vi "UHR-Fleezers Control (host) - 10.7.vi"() -> ()   [LabVIEW 2010] (continued)
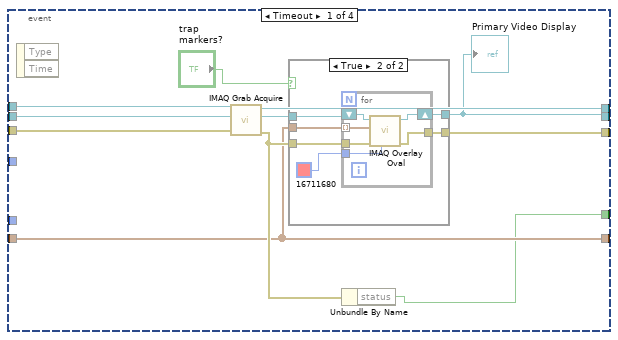
[diagram p2: hidden frame]
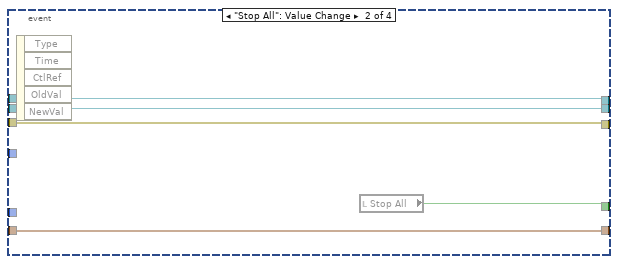
[diagram p4: hidden frame]
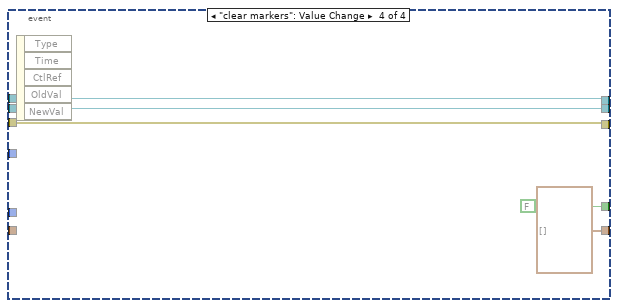
[diagram p6: hidden frame]
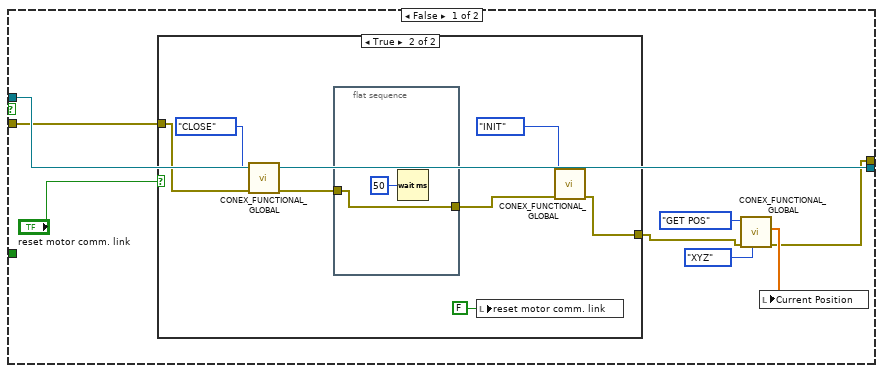
[diagram p8: hidden frame]
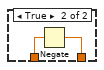
[diagram p12: hidden frame]
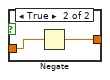
[diagram p13: hidden frame]
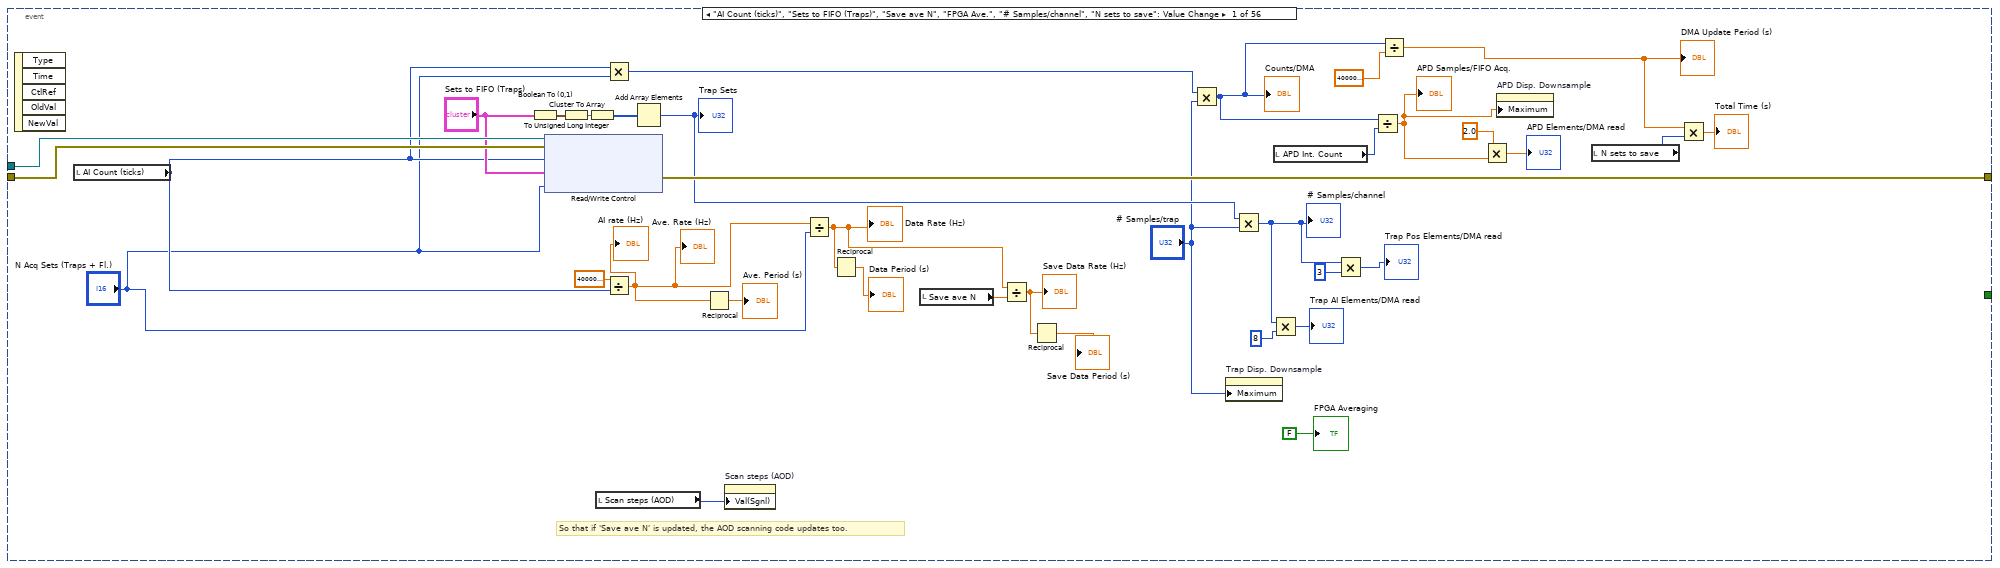
[diagram p14: hidden frame]
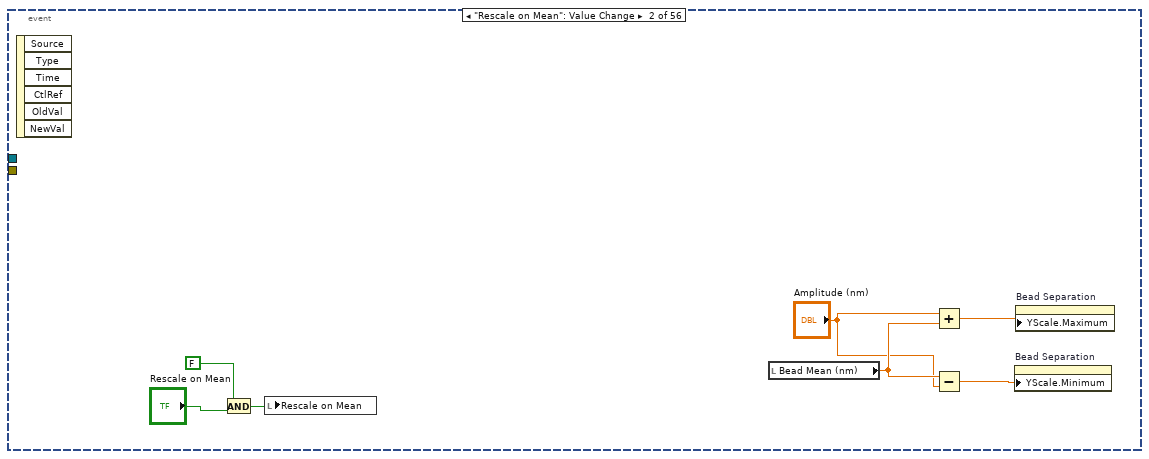
[diagram p15: hidden frame]
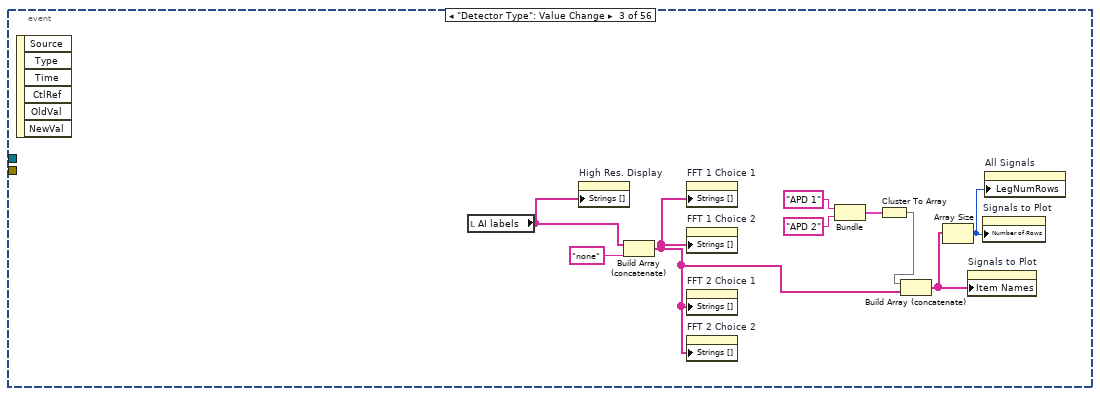
[diagram p16: hidden frame]
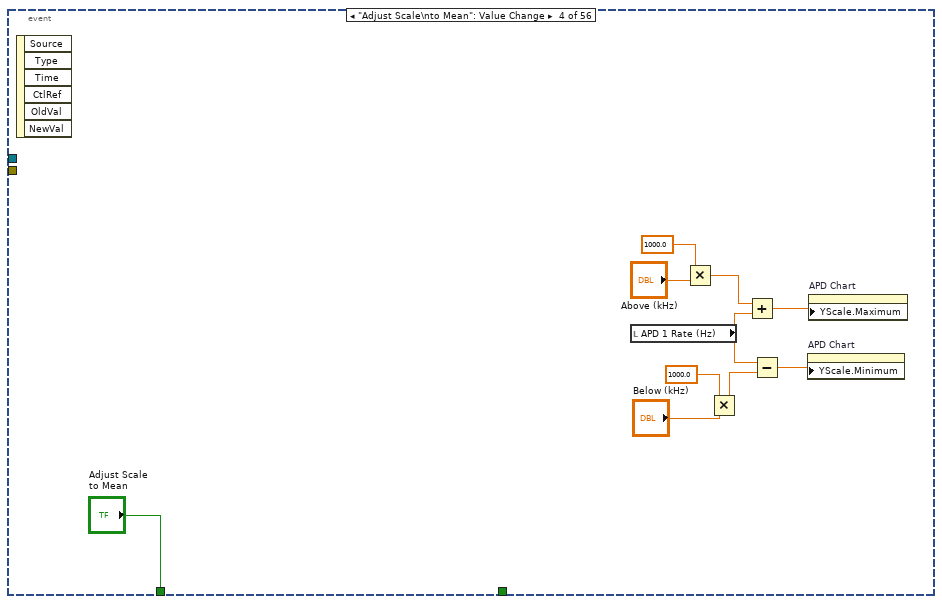
[diagram p17: hidden frame]
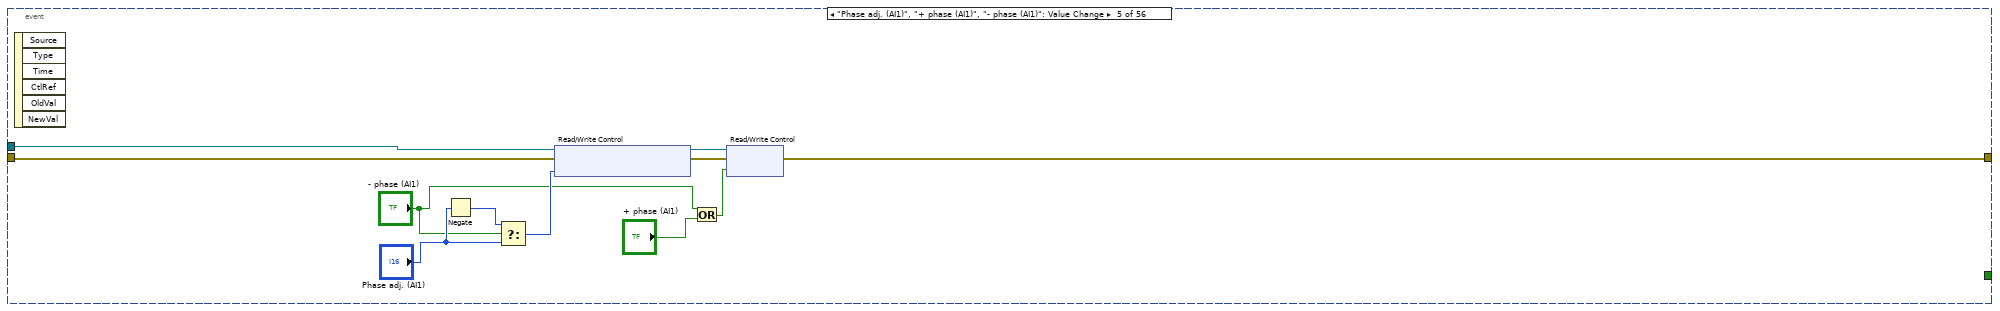
[diagram p18: hidden frame]
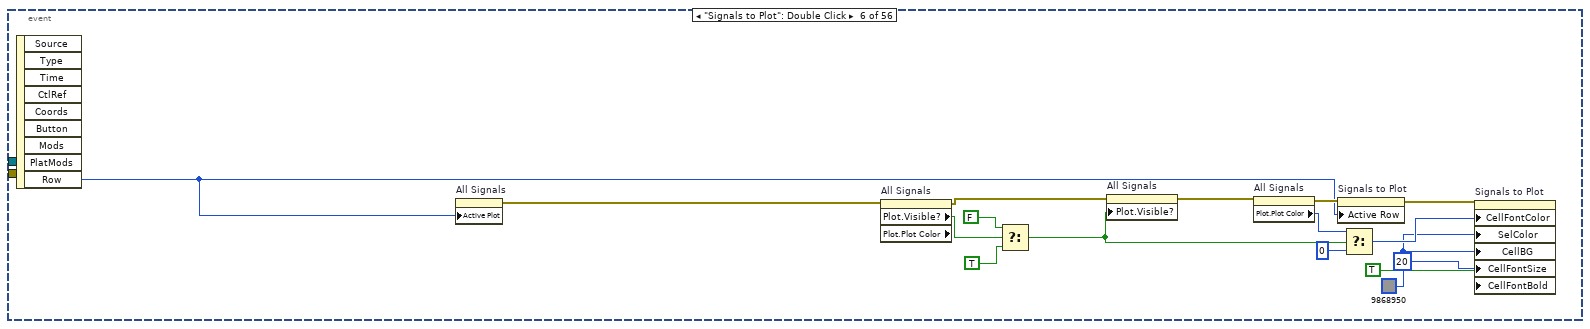
[diagram p19: hidden frame]
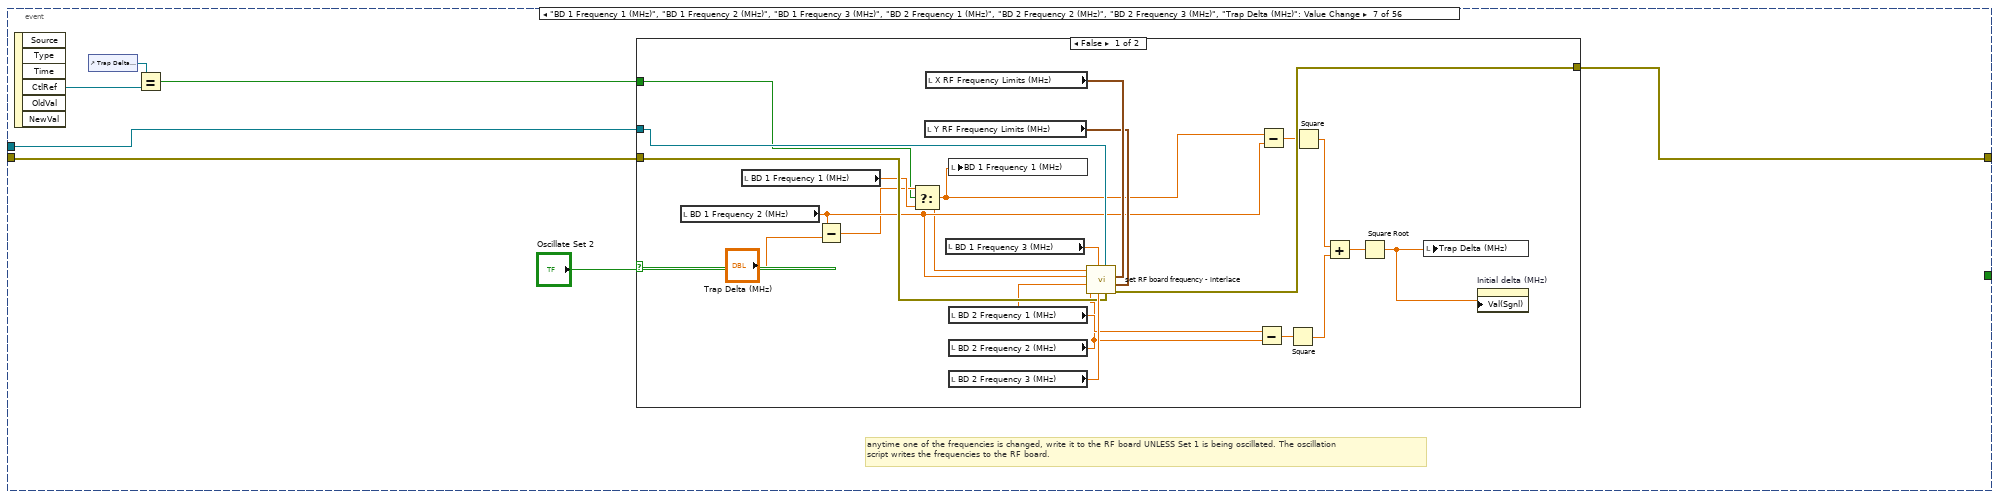
[diagram p20: hidden frame]
                n2083 = Divide "X half step offset"(x=w8714, y=2.0) -> (x/y=w8724:dbl)
                n2084 = Divide "X V/pix"(x=w8714, y=w8727) -> (x/y=w8726:dbl)
                n2085 = Multiply(x=w8714, y=w8721) -> (x*y=w8733:dbl)
                n2086 = Compound Arithmetic op=ADD(w8731, w8738, w8737) -> (w8715:dbl)
                "Pointer Y (V)" <- w8715
                n2087 = Multiply(x=w8726, y=w8720) -> (x*y=w8735:dbl)
                n2088 = Negate(x=w8724) -> (-x=w8723:dbl)
                n2089 = local read "Initial X"() -> (w8736:dbl)
                n2090 = Negate(x=w8735) -> (-x=w8734:dbl)
                n2091 = Compound Arithmetic op=ADD(w8723, w8733, w8736, w8734) -> (w8716:dbl)
                "Pointer X (V)" <- w8716
                n2092 = Or(x="Set X Only", y="Set Confocal Spot (X-Y)") -> (x .or. y?=w8709:bool)
                n2093 = Or(x="Set Confocal Spot (X-Y)", y="Set Y Only") -> (x .or. y?=w8708:bool)
                n2094 = case shown="True" w8709 {
                  tunnel: w8716 -> [_ w8739]
                  frame False {
                  }
                  frame True {
                    n2095 = property on="AO2" class="Slide (strict)"("Val(Sgnl)"=w8739) -> ()  [unwired: 2 in, 2 out]
                  }
                }
                n2096 = case shown="True" w8708 {
                  tunnel: w8715 -> [_ w8740]
                  frame False {
                  }
                  frame True {
                    n2097 = property on="AO1" class="Slide (strict)"("Val(Sgnl)"=w8740) -> ()  [unwired: 2 in, 2 out]
                  }
                }
                n2098 = local write "Set Confocal Spot (X-Y)"(w8713) -> ()
                n2099 = local write "Set X Only"(w8713) -> ()
                n2100 = local write "Set Y Only"(w8713) -> ()
              }
            }
          }
          frame 3 {
            n2101 = local read "BD 2 Frequency 1 (MHz)"() -> (w8741:dbl)
            n2102 = local read "BD 1 Frequency 1 (MHz)"() -> (w8742:dbl)
            n2103 = local write "Manipulating Trap"(TRUE ("Manipulating Trap")) -> ()
            n2104 = local write "Coords"(T7 {"Horizontal"=0, "Vertical"=0} ("Coords")) -> ()
            n2105 = while {
              tunnel: w8747 -> [w8752]
              tunnel: w8745 -> [w8751]
              tunnel: w8743 -> [w8750]
              tunnel: w8742 -> [w8749]
              tunnel: w8741 -> [w8748]
              stop <- w8753 stop-if-true
              n2106 = event shown="[0] \"Pane\": Mouse Move" {
                selector: _ -> [_ _]
                dyn-events: _ -> [_ _]
                timeout: _ -> [_ _]
                tunnel: ["Force Manip Abort" w8817] -> w8753
                tunnel: w8752 -> [w8760 _]
                tunnel: w8751 -> [w8758 _]
                tunnel: w8750 -> [w8757 _]
                tunnel: w8749 -> [w8756 _]
                tunnel: w8748 -> [w8755 _]
                event Mouse Move {
                  n2107 = event-data() -> ("Time"=w8761:u32, "Coords"=w8762:T7)  [unwired: 3 out]
                  n2108 = Less?(x=w8761, y=w8760) -> (x < y?=w8759:bool)
                  n2109 = case "Makes sure old motion events prior to mouse click aren't used" shown="False" w8759 {
                    tunnel: w8762 -> [w8804 _]
                    tunnel: w8758 -> [w8805 _]
                    tunnel: w8757 -> [w8782 _]
                    tunnel: w8756 -> [w8778 _]
                    tunnel: w8755 -> [w8777 _]
                    frame False {
                      n2110 = Subtract(x=w8804, y=w8805) -> (x-y=w8803:T7)
                      "Coords" <- w8803
                      n2111 = local read "Y RF Frequency Limits (MHz)"() -> (w8763:T16)
                      n2112 = To Double Precision Float(number=w8803) -> (double precision float=w8802:cluster{"Horizontal":dbl, "Vertical":dbl})
                      n2113 = Multiply(x=cluster{"Horizontal":dbl, "Vertical":dbl} {"Horizontal"=-1.0, "Vertical"=1.0}, y="Manipulation Scaling") -> (x*y=w8798:cluster{"Horizontal":dbl, "Vertical":dbl})
                      n2114 = local read "X RF Frequency Limits (MHz)"() -> (w8764:T16)
                      n2115 = Multiply(x=w8802, y=w8798) -> (x*y=w8800:cluster{"Horizontal":dbl, "Vertical":dbl})
                      n2116 = Unbundle By Name(w8800) -> ("Horizontal"=w8795:dbl, "Vertical"=w8799:dbl)
                      n2117 = Unbundle By Name(w8763) -> ("Maximum"=w8766:dbl, "Minimum"=w8765:dbl)
                      n2118 = Boolean To (0,1)(Boolean="Manip. X?") -> (0, 1=w8793:i16)
                      n2119 = Boolean To (0,1)(Boolean="Manip. Y?") -> (0, 1=w8790:i16)
                      n2120 = local read "BD 1 Frequency 2 (MHz)"() -> (w8780:dbl)
                      n2121 = Multiply(x=w8799, y=w8790) -> (x*y=w8792:dbl)
                      n2122 = Multiply(x=w8793, y=w8795) -> (x*y=w8796:dbl)
                      n2123 = local read "BD 2 Frequency 2 (MHz)"() -> (w8779:dbl)
                      n2124 = Unbundle By Name(w8764) -> ("Maximum"=w8768:dbl, "Minimum"=w8767:dbl)
                      n2125 = Add(x=w8777, y=w8792) -> (x+y=w8770:dbl)
                      n2126 = Add(x=w8778, y=w8796) -> (x+y=w8772:dbl)
                      n2127 = In Range and Coerce(upper limit=w8768, x=w8772, lower limit=w8767) -> (coerced(x)=w8771:dbl)  [unwired: 1 out]
                      n2128 = In Range and Coerce(upper limit=w8766, x=w8770, lower limit=w8765) -> (coerced(x)=w8769:dbl)  [unwired: 1 out]
                      n2129 = Subtract(x=w8771, y=w8780) -> (x-y=w8789:dbl)
                      n2130 = Subtract(x=w8769, y=w8779) -> (x-y=w8788:dbl)
                      n2131 = Square(x=w8789) -> (x^2=w8787:dbl)
                      n2132 = Square(x=w8788) -> (x^2=w8786:dbl)
                      n2133 = Add(x=w8787, y=w8786) -> (x+y=w8785:dbl)
                      n2134 = Square Root(x=w8785) -> (sqrt(x)=w8781:dbl)
                      n2135 = In Range and Coerce(upper limit="Limit Max (MHz)", x=w8781, lower limit="Limit Min (MHz)") -> (In Range?=w8774:bool)  [unwired: 1 out]
                      n2136 = Not(x="Limits Enable") -> (.not. x?=w8773:bool)
                      n2137 = Or(x=w8774, y=w8773) -> (x .or. y?=w8775:bool)
                      n2138 = case shown="True" w8775 {
                        tunnel: w8782 -> [_ w8815]
                        tunnel: w8781 -> [_ w8806]
                        tunnel: w8771 -> [_ w8813]
                        tunnel: w8780 -> [_ w8812]
                        tunnel: w8769 -> [_ w8811]
                        tunnel: w8779 -> [_ w8810]
                        tunnel: w8764 -> [_ w8808]
                        tunnel: w8763 -> [_ w8807]
                        frame False {
                        }
                        frame True {
                          n2139 = local read "BD 1 Frequency 3 (MHz)"() -> (w8814:dbl)
                          n2140 = local read "BD 2 Frequency 3 (MHz)"() -> (w8809:dbl)
                          n2141 = local write "Trap Delta (MHz)"(w8806) -> ()
                          n2142 = property on="Initial delta (MHz)" class="DigNum (strict)"("Val(Sgnl)"=w8806) -> ()  [unwired: 2 in, 2 out]
                          n2143 = call "set RF board frequency - interlace.vi"("Board 2 Frequency Limits"=w8807, "Board 1 Frequency Limits"=w8808, "FPGA VI Reference In"=w8815, "Board 2 Frequency 3 (MHz)"=w8809, "Board 1 Frequency 3 (MHz)"=w8814, "Board 2 Frequency 2 (MHz)"=w8810, "Board 2 Frequency 1 (MHz)"=w8811, "Board 1 Frequency 2 (MHz)"=w8812, "Board 1 Frequency 1  (MHz)"=w8813) -> ()  [unwired: 1 in, 2 out]
                          n2144 = local write "BD 2 Frequency 1 (MHz)"(w8811) -> ()
                          n2145 = local write "BD 1 Frequency 1 (MHz)"(w8813) -> ()
                        }
                      }
                    }
                    frame True {
                    }
                  }
                }
                event Mouse Up {
                  n2146 = event-data() -> ("Button"=w8816:u16)  [unwired: 8 out]
                  n2147 = case shown="3" w8816 {
                    tunnel: [FALSE TRUE] -> w8817
                    frame 0, Default {
                    }
                    frame 3 {
                      n2148 = local write "Manipulating Trap"(FALSE ("Manipulating Trap")) -> ()
                    }
                  }
                }
              }
            }
          }
        }
      }
      event Mouse Move {
        n2149 = event-data() -> ()  [unwired: 6 out]
      }
    }
    n2150 = local read "Stop All"() -> (w8638:bool)
    n2151 = node-c288() -> ()  [unwired: 2 out]
  }
  n2152 = timed-loop "Oscillate AOD (debugging)" {
    tunnel: w16 -> [w8822]
    tunnel: [w8821] -> w33
    timing: w73 -> [_]
    timing-out: [_] -> w72
    stop <- w8821 stop-if-true
    n2153 = node-c288() -> ()  [unwired: 2 out]
    n2154 = event shown="[0] \"Oscillate Set 2\", \"Fish for Tether\": Value Change" {
      selector: _ -> [_ _ _]
      dyn-events: _ -> [_ _ _]
      timeout: _ -> [_ _ _]
      tunnel: w8822 -> [w8829 _ _]
      tunnel: [FALSE ("Stop All") _ w9098] -> w8821
      event "Oscillate Set 2", "Fish for Tether": Value Change {
        n2155 = event-data() -> ()  [unwired: 6 out]
        n2156 = local read "Oscillate Set 2"() -> (w8828:bool)
        n2157 = Or(x=w8828, y="Fish for Tether") -> (x .or. y?=w8826:bool)
        n2158 = case shown="True" w8826 {
          tunnel: w8829 -> [_ w8832]
          tunnel: "Fish for Tether" -> [_ w8831]
          frame False {
          }
          frame True {
            n2159 = case shown="True" w8831 {
              frame False {
              }
              frame True {
                n2160 = local write "Scan axis 2"(TRUE) -> ()
                n2161 = local write "Tether"(FALSE ("Tether")) -> ()
              }
            }
            n2162 = node-c288("Period") -> (w8834:T26)  [unwired: 3 out]
            n2163 = timed-loop "Oscillate AOD" {
              timing: w8834 -> [_]
              timing-out: [_] -> w8833
              tunnel: w8832 -> [w8844]
              tunnel: w8831 -> [w8843]
              i -> [w8846]
              stop <- w8842 stop-if-true
              n2164 = node-c288() -> (w8845:i64)  [unwired: 1 out]
              n2165 = flat-sequence {
                tunnel: w8846 -> [w8873]
                tunnel: w8845 -> [w8872]
                tunnel: w8844 -> [w8854]
                tunnel: w8843 -> [w8856]
                tunnel: [w8856] -> w8841
                tunnel: [w8855] -> w8840
                tunnel: [w8853] -> w8839
                tunnel: [w8850] -> w8837
                tunnel: w8841 -> [w8909]
                tunnel: w8840 -> [w8907]
                tunnel: w8839 -> [w8906]
                tunnel: [w8905] -> w8838
                tunnel: w8837 -> [w8904]
                tunnel: [w8973] -> w8842
                tunnel: w8838 -> [w8971]
                frame #0 {
                  n2166 = Divide(x=w8872, y=i64 1000) -> (x/y=w8867:dbl)
                  n2167 = Multiply(x=w8867, y=w8873) -> (x*y=w8869:dbl)
                  n2168 = Multiply(x="Osc. freq. (Hz)", y=6.283185307179586) -> (x*y=w8870:dbl)
                  n2169 = Multiply(x=w8870, y=w8869) -> (x*y=w8852:dbl)
                  n2170 = local read "BD 1 Frequency 2 (MHz)"() -> (w8847:dbl)
                  n2171 = local read "BD 1 Frequency 1 (MHz)"() -> (w8848:dbl)
                  n2172 = case shown="True" w8856 {
                    tunnel: w8852 -> [w8879 w8885]
                    tunnel: w8847 -> [_ w8896]
                    tunnel: [w8876 w8891] -> w8857
                    tunnel: [FALSE w8888] -> w8853
                    tunnel: [0.0 w8881] -> w8850
                    tunnel: w8848 -> [_ w8880]
                    frame False {
                      n2173 = Sine(x=w8879) -> (sin(x)=w8877:dbl)
                      n2174 = Multiply(x=w8877, y="Osc. amp. (MHz)") -> (x*y=w8876:dbl)
                    }
                    frame True {
                      n2175 = Cosine(x=w8885) -> (cos(x)=w8899:dbl)
                      n2176 = Subtract(x=w8896, y=w8880) -> (x-y=w8895:dbl)
                      n2177 = Decrement(x=w8899) -> (x-1=w8898:dbl)
                      n2178 = Subtract(x=w8895, y="Closest Delta (MHz)") -> (x-y=w8892:dbl)
                      n2179 = Divide(x=w8898, y=-2.0) -> (x/y=w8893:dbl)
                      n2180 = Multiply(x=w8893, y=w8892) -> (x*y=w8891:dbl)
                      n2181 = local read "Vec Mean of T1 T2"() -> (w8887:dbl[])
                      n2182 = Greater?(x=w8887, y="Stop F (pN)") -> (0:w8889:bool[])
                      n2183 = Or Array Elements(Boolean array=w8889) -> (logical OR=w8888:bool)
                      n2184 = Divide(x=w8885, y=6.283185307179586) -> (x/y=w8884:dbl)
                      n2185 = Round Toward +Infinity(x=w8884) -> (ceil(x): smallest int >= x=w8881:dbl)
                      "Attempts" <- w8881
                      n2186 = Greater?(x=w8881, y="Attempt Limit") -> (0:w8883:bool)
                      n2187 = case shown="True" w8883 {
                        frame False {
                        }
                        frame True {
                          n2188 = local write "Fish for Tether"(FALSE ("Fish for Tether")) -> ()
                          n2189 = call <vilib>:"Beep.vi"() -> ()  [unwired: 3 in, 9 out]
                          n2190 = local read "Messages"() -> (w8901:string)
                          n2191 = call "Update messages.vi"("Message to add"="Tether fishing timeout." ("Messages"), "Old message string"=w8901) -> ("New message string"=→"Messages":string)
                        }
                      }
                    }
                  }
                  n2192 = local read "BD 2 Frequency 1 (MHz)"() -> (w8858:dbl)
                  n2193 = Select(t=w8848, s="Scan axis 2", f=w8858) -> (s? t:f=w8861:dbl)
                  n2194 = Add(x=w8857, y=w8861) -> (x+y=w8855:dbl)
                  n2195 = Select(t=w8855, s="Scan axis 2", f=w8848) -> (s? t:f=w8849:dbl)
                  n2196 = Select(t=w8858, s="Scan axis 2", f=w8855) -> (s? t:f=w8863:dbl)
                  n2197 = local read "Y RF Frequency Limits (MHz)"() -> (w8859:T16)
                  n2198 = local read "X RF Frequency Limits (MHz)"() -> (w8860:T16)
                  n2199 = local read "BD 1 Frequency 3 (MHz)"() -> (w8866:dbl)
                  n2200 = local read "BD 2 Frequency 2 (MHz)"() -> (w8865:dbl)
                  n2201 = local read "BD 2 Frequency 3 (MHz)"() -> (w8864:dbl)
                  n2202 = call "set RF board frequency - interlace.vi"("Board 2 Frequency Limits"=w8859, "Board 1 Frequency Limits"=w8860, "FPGA VI Reference In"=w8854, "Board 2 Frequency 3 (MHz)"=w8864, "Board 1 Frequency 3 (MHz)"=w8866, "Board 2 Frequency 2 (MHz)"=w8865, "Board 2 Frequency 1 (MHz)"=w8863, "Board 1 Frequency 2 (MHz)"=w8847, "Board 1 Frequency 1  (MHz)"=w8849) -> ()  [unwired: 1 in, 2 out]
                }
                frame #1 {
                  n2203 = And(x=w8909, y=w8906) -> (x .and. y?=w8908:bool)
                  n2204 = case "Only if were fishing and now formed tether" shown="False" w8908 {
                    tunnel: w8907 -> [w8911 w8923]
                    tunnel: [w8910 w8922] -> w8905
                    tunnel: w8904 -> [_ w8918]
                    frame False {
                      n2205 = local read "Fish for Tether"() -> (w8910:bool)
                      n2206 = case shown="True" w8910 {
                        tunnel: w8911 -> [_ _]
                        frame False {
                        }
                        frame True {
                        }
                      }
                    }
                    frame True {
                      w8922 = FALSE ("Fish for Tether")
                      n2207 = call <vilib>:"Beep.vi"() -> ()  [unwired: 3 in, 9 out]
                      n2208 = Number To Decimal String(number=w8918, width (-)=i16 1) -> (decimal integer string=w8916:string)
                      n2209 = case shown="\"1\", Default" "Then..." {
                        selector: "Then..." -> [_ w8926]
                        tunnel: w8923 -> [w8925 _]
                        frame "1", Default {
                          n2210 = property on="BD 1 Frequency 1 (MHz)" class="DigNum (strict)"("Val(Sgnl)"=w8925) -> ()  [unwired: 2 in, 2 out]
                        }
                        frame "2", "3", "4", "5", "6" {
                          n2211 = flat-sequence {
                            tunnel: w8926 -> [w8928]
                            frame #0 {
                              n2212 = property on="Trap Delta (MHz)" class="DigNum (strict)"("Val(Sgnl)"="Move to Delta 1 (MHz)") -> ()  [unwired: 2 in, 2 out]
                            }
                            frame #1 {
                              n2213 = case shown="\"5\", \"6\"" w8928 {
                                selector: w8928 -> [w8931 w8941 _]
                                frame "3", "4" {
                                n2214 = flat-sequence {
                                tunnel: w8931 -> [w8932]
                                tunnel: [w8932] -> w8929
                                tunnel: [w8934] -> w8930
                                tunnel: w8929 -> [w8934]
                                tunnel: w8930 -> [w8938]
                                frame #0 {
                                n2215 = property on="Green Laser ON/Interlacing" class="Bool (strict)"("Val(Sgnl)"=TRUE ("Value (Signaling)")) -> ()  [unwired: 2 in, 2 out]
                                }
                                frame #1 {
                                n2216 = Multiply(x="Wait Before Save (s)", y=u32 1000 ("x")) -> (x*y=w8936:u32)
                                n2217 = Wait (ms)(milliseconds to wait=w8936) -> ()  [unwired: 1 out]
                                }
                                frame #2 {
                                n2218 = property on="Start Saving" class="Bool (strict)"("Value"=TRUE ("Start Saving")) -> ()  [unwired: 2 in, 2 out]
                                n2219 = case shown="\"4\"" w8938 {
                                frame Default {
                                }
                                frame "4" {
                                n2220 = property on="Fl. Triggered..." class="Bool (strict)"("Val(Sgnl)"=TRUE ("Value (Signaling)")) -> ()  [unwired: 2 in, 2 out]
                                }
                                }
                                }
                                }
                                }
                                frame "5", "6" {
                                n2221 = stacked-sequence {
                                tunnel: w8941 -> [_ _ _ _ _ _ _ _ w8958 _ _]
                                frame #0 {
                                n2222 = Replace Array Subset(array=u32[] [0] ("Index Values"), new element="Raster Set Upon Tether", index=0) -> (w8942:u32[])
                                n2223 = property on="Saved AOD Raster Scan Parameter Sets" class="Arr (strict)"("Index Values"=w8942) -> ()  [unwired: 2 in, 2 out]
                                }
                                frame #1 {
                                n2224 = Wait (ms)(milliseconds to wait=u32 500) -> ()  [unwired: 1 out]
                                }
                                frame #2 {
                                n2225 = property on="Load parameters" class="Bool (strict)"("Val(Sgnl)"=TRUE ("Value (Signaling)")) -> ()  [unwired: 2 in, 2 out]
                                }
                                frame #3 {
                                n2226 = Wait (ms)(milliseconds to wait=u32 500) -> ()  [unwired: 1 out]
                                }
                                frame #4 {
                                n2227 = property on="Trap Raster Scan" class="Bool (strict)"("Val(Sgnl)"=TRUE ("Value (Signaling)")) -> ()  [unwired: 2 in, 2 out]
                                }
                                frame #5 {
                                n2228 = Wait (ms)(milliseconds to wait=u32 2000) -> ()  [unwired: 1 out]
                                }
                                frame #6 {
                                n2229 = while {
                                stop <- w8953 stop-if-true
                                n2230 = local read "Raster Scanning..."() -> (w8952:bool)
                                n2231 = local read "Saving..."() -> (w8955:bool)
                                n2232 = Wait (ms)(milliseconds to wait=u32 100) -> ()  [unwired: 1 out]
                                n2233 = Not(x=w8955) -> (.not. x?=w8954:bool)
                                n2234 = Not(x=w8952) -> (.not. x?=w8951:bool)
                                n2235 = And(x=w8954, y=w8951) -> (x .and. y?=w8953:bool)
                                }
                                }
                                frame #7 {
                                n2236 = property on="Trap Delta (MHz)" class="DigNum (strict)"("Val(Sgnl)"="Move to Delta 2 (MHz)") -> ()  [unwired: 2 in, 2 out]
                                }
                                frame #8 {
                                n2237 = local read "Tether"() -> (w8959:bool)
                                n2238 = case shown="True" w8959 {
                                tunnel: w8958 -> [_ w8960]
                                frame False {
                                }
                                frame True {
                                n2239 = flat-sequence {
                                tunnel: w8960 -> [w8962]
                                frame #0 {
                                n2240 = Wait (ms)(milliseconds to wait=u32 500) -> ()  [unwired: 1 out]
                                }
                                frame #1 {
                                n2241 = case shown="\"6\"" w8962 {
                                frame Default {
                                }
                                frame "6" {
                                n2242 = property on="Green Laser ON/Interlacing" class="Bool (strict)"("Val(Sgnl)"=TRUE ("Green Laser ON/Interlacing")) -> ()  [unwired: 2 in, 2 out]
                                }
                                }
                                }
                                frame #2 {
                                n2243 = Wait (ms)(milliseconds to wait=u32 500) -> ()  [unwired: 1 out]
                                }
                                frame #3 {
                                n2244 = local write "Start Saving"("Save at end (5, 6)") -> ()
                                }
                                }
                                }
                                }
                                }
                                frame #9 {
                                n2245 = local read "Bead Sep. Int. Time (s)"() -> (w8968:dbl)
                                n2246 = Multiply(x=w8968, y=1000.0) -> (x*y=w8967:dbl)
                                n2247 = Wait (ms)(milliseconds to wait=w8967) -> ()  [unwired: 1 out]
                                }
                                frame #10 {
                                n2248 = property on="Rescale on Mean" class="Bool (strict)"("Val(Sgnl)"=TRUE ("Value (Signaling)")) -> ()  [unwired: 2 in, 2 out]
                                }
                                }
                                }
                                frame "2", Default {
                                }
                              }
                            }
                          }
                        }
                      }
                      n2249 = Concatenate Strings("Formed tether in ", w8916, " attempt(s)." ("string")) -> (w8913:string)
                      n2250 = local read "Messages"() -> (w8920:string)
                      n2251 = local write "Fish for Tether"(w8922) -> ()
                      n2252 = call "Update messages.vi"("Message to add"=w8913, "Old message string"=w8920) -> ("New message string"=w8919:string)
                      n2253 = local write "Messages"(w8919) -> ()
                      n2254 = Get Date/Time In Seconds() -> (seconds since 1Jan1904=→"Time tether formed":timestamp)
                      "Tether" <- "Tether Alarm?"
                    }
                  }
                }
                frame #2 {
                  n2255 = local read "Oscillate Set 2"() -> (w8972:bool)
                  n2256 = local read "Stop All"() -> (w8974:bool)
                  n2257 = Not Or(1:w8971, 2:w8972) -> (0:w8970:bool)
                  n2258 = Compound Arithmetic op=OR(w8974, w8970) -> (w8973:bool)
                }
              }
              n2259 = node-c288() -> ()  [unwired: 2 out]
            }
            n2260 = node-c288(w8833) -> ()  [unwired: 1 out]
          }
        }
      }
      event "Fl. Triggered...": Value Change {
        n2261 = event-data() -> ()  [unwired: 7 out]
        n2262 = case shown="True" "Fl. Triggered..." {
          frame False {
          }
          frame True {
            n2263 = node-c288() -> (w8986:T26)  [unwired: 4 out]
            n2264 = timed-loop {
              timing: w8986 -> [_]
              timing-out: [_] -> w8985
              tunnel: "Action" -> [w8990]
              shift-right: [w8987] -> _
              shift-left: u8 255 -> [w8989]
              stop <- w8991 stop-if-true
              n2265 = node-c288() -> ()  [unwired: 2 out]
              n2266 = flat-sequence {
                tunnel: w8990 -> [w9003]
                tunnel: w8989 -> [w9000]
                tunnel: [w8999] -> w8988
                tunnel: [w9089] -> w8991
                tunnel: w8988 -> [w9088]
                tunnel: [w9088] -> w8987
                frame #0 {
                  n2267 = local read "Delta Fl. 2"() -> (w8994:dbl)
                  n2268 = local read "Delta Fl. 1"() -> (w8995:dbl)
                  n2269 = Select(t=w8995, s="APD to Watch", f=w8994) -> (s? t:f=w8993:dbl)
                  n2270 = Multiply(x="Fl. Delta Thresh. (kHz)", y=1000.0) -> (x*y=w9002:dbl)
                  n2271 = Greater?(x=w8993, y=w9002) -> (0:w8997:bool)
                  n2272 = Or(x="Force Yank", y=w8997) -> (x .or. y?=w8998:bool)
                  n2273 = case shown="True" w8998 {
                    tunnel: w9003 -> [_ w9013]
                    tunnel: w9000 -> [w9005 w9009]
                    tunnel: [w9005 w9006] -> w8999
                    frame False {
                    }
                    frame True {
                      n2274 = flat-sequence {
                        tunnel: w9010 -> [w9019]
                        tunnel: [w9019] -> w9014
                        tunnel: w9013 -> [w9018]
                        tunnel: [w9018] -> w9012
                        tunnel: [w9017] -> w9011
                        tunnel: w9009 -> [w9016]
                        tunnel: [w9015] -> w9008
                        tunnel: w9014 -> [w9044]
                        tunnel: w9012 -> [w9043]
                        tunnel: w9011 -> [w9042]
                        tunnel: w9008 -> [w9041]
                        tunnel: [w9041] -> w9007
                        tunnel: w9007 -> [w9086]
                        tunnel: [w9086] -> w9006
                        frame #0 {
                          n2275 = call <vilib>:"Beep.vi"() -> ()  [unwired: 3 in, 9 out]
                          n2276 = local write "Waiting"(FALSE ("Waiting")) -> ()
                          n2277 = Increment(x=w9016) -> (x+1=w9015:u8)
                          n2278 = case shown="\"Yank\"" w9018 {
                            tunnel: w9015 -> [_ _ w9025]
                            frame "Image" {
                              n2279 = property on="Confocal Image" class="Bool (strict)"("Val(Sgnl)"=TRUE ("Value (Signaling)")) -> ()  [unwired: 2 in, 2 out]
                            }
                            frame "Alarm", Default {
                            }
                            frame "Yank" {
                              n2280 = flat-sequence {
                                tunnel: w9025 -> [w9028]
                                tunnel: [w9027] -> w9024
                                tunnel: ["N Array El"] -> w9023
                                tunnel: w9024 -> [w9038]
                                tunnel: w9023 -> [w9034]
                                frame #0 {
                                n2281 = Multiply(x="Yank Delay (s)", y=1000.0) -> (x*y=w9031:dbl)
                                n2282 = Quotient & Remainder(x=w9028, y="N Array El") -> (x-y*floor(x/y)=w9027:u8)  [unwired: 1 out]
                                n2283 = Wait (ms)(milliseconds to wait=w9031) -> ()  [unwired: 1 out]
                                }
                                frame #1 {
                                n2284 = Random Number (0-1)() -> (number: 0 to 1=w9035:dbl)
                                n2285 = Multiply(x=w9034, y=w9035) -> (x*y=w9033:dbl)
                                n2286 = Round Toward -Infinity(1:w9033) -> (0:w9032:dbl)
                                n2287 = Select(t=w9032, s="Random Choice", f=w9038) -> (s? t:f=w9036:dbl)
                                n2288 = Index Array(array="Yank to Delta Array (MHz)", index=w9036) -> (element=w9039:dbl)
                                n2289 = property on="Trap Delta (MHz)" class="DigNum (strict)"("Val(Sgnl)"=w9039) -> ()  [unwired: 2 in, 2 out]
                                }
                              }
                            }
                          }
                          n2290 = local read "Time (s)"() -> (w9017:dbl)
                          "Fl. High" <- TRUE ("Yanking")
                        }
                        frame #1 {
                          n2291 = node-c288() -> (w9046:T26)  [unwired: 4 out]
                          n2292 = timed-loop {
                            timing: w9046 -> [_]
                            timing-out: [_] -> w9045
                            tunnel: w9044 -> [w9062]
                            tunnel: w9043 -> [w9060]
                            tunnel: w9042 -> [w9059]
                            stop <- w9061 stop-if-true
                            n2293 = node-c288() -> ()  [unwired: 2 out]
                            n2294 = local read "Fl. Delta Thresh. (kHz)"() -> (w9054:dbl)
                            n2295 = local read "Fl. Triggered..."() -> (w9063:bool)
                            n2296 = local read "Delta Fl. 1"() -> (w9050:dbl)
                            n2297 = local read "Delta Fl. 2"() -> (w9048:dbl)
                            n2298 = local read "Stop All"() -> (w9057:bool)
                            n2299 = local read "APD to Watch"() -> (w9049:bool)
                            n2300 = Select(t=w9050, s=w9049, f=w9048) -> (s? t:f=w9047:dbl)
                            n2301 = Not(x=w9063) -> (.not. x?=w9058:bool)
                            n2302 = Multiply(x=w9054, y=1000.0) -> (x*y=w9053:dbl)
                            n2303 = Negate(x=w9053) -> (-x=w9052:dbl)
                            n2304 = Less?(x=w9047, y=w9052) -> (x < y?=w9056:bool)
                            n2305 = Compound Arithmetic op=OR(w9056, w9057, w9058, "Force Reset") -> (w9061:bool)
                            n2306 = case shown="True" w9061 {
                              tunnel: w9062 -> [_ w9074]
                              tunnel: w9060 -> [_ w9073]
                              tunnel: w9059 -> [_ w9071]
                              frame False {
                              }
                              frame True {
                                n2307 = case shown="\"Yank\"" w9073 {
                                tunnel: w9074 -> [_ w9075]
                                frame "Image", Default {
                                }
                                frame "Yank" {
                                n2308 = flat-sequence {
                                tunnel: [w9080] -> w9076
                                tunnel: w9075 -> [w9080]
                                tunnel: w9076 -> [w9081]
                                frame #0 {
                                n2309 = local read "Yank Delay (s)"() -> (w9079:dbl)
                                n2310 = Multiply(x=w9079, y=1000.0) -> (x*y=w9077:dbl)
                                n2311 = Wait (ms)(milliseconds to wait=w9077) -> ()  [unwired: 1 out]
                                }
                                frame #1 {
                                n2312 = property on="Trap Delta (MHz)" class="DigNum (strict)"("Val(Sgnl)"=w9081) -> ()  [unwired: 2 in, 2 out]
                                }
                                }
                                }
                                }
                                n2313 = local read "Time (s)"() -> (w9072:dbl)
                                n2314 = Subtract(x=w9072, y=w9071) -> (x-y=w9068:dbl)
                                "Duration (s)" <- w9068
                                n2315 = Number To Decimal String(number=w9068, width (-)=i16 0) -> (decimal integer string=w9066:string)
                                n2316 = Concatenate Strings(w9066, " s fluorescence event." ("string")) -> (w9064:string)
                                n2317 = local read "Messages"() -> (w9070:string)
                                n2318 = call "Update messages.vi"("Message to add"=w9064, "Old message string"=w9070) -> ("New message string"=w9069:string)
                                n2319 = call <vilib>:"Beep.vi"() -> ()  [unwired: 3 in, 9 out]
                                n2320 = local write "Messages"(w9069) -> ()
                              }
                            }
                            n2321 = node-c288() -> ()  [unwired: 2 out]
                          }
                          n2322 = node-c288(w9045) -> ()  [unwired: 1 out]
                        }
                        frame #2 {
                          n2323 = local write "Fl. High"(FALSE ("Yanking")) -> ()
                        }
                      }
                      n2324 = local read "Trap Delta (MHz)"() -> (w9010:dbl)
                    }
                  }
                }
                frame #1 {
                  n2325 = local read "Stop All"() -> (w9092:bool)
                  n2326 = local read "Fl. Triggered..."() -> (w9090:bool)
                  n2327 = Not(x=w9090) -> (.not. x?=w9091:bool)
                  n2328 = Or(x=w9091, y=w9092) -> (x .or. y?=w9089:bool)
                  n2329 = Not(x=w9089) -> (.not. x?=→"Waiting":bool)
                }
              }
              n2330 = node-c288() -> ()  [unwired: 2 out]
            }
            n2331 = node-c288(w8985) -> ()  [unwired: 1 out]
          }
        }
      }
      event "Stop All": Value Change {
        n2332 = event-data() -> ()  [unwired: 7 out]
        n2333 = local read "Stop All"() -> (w9098:bool)
      }
    }
    n2334 = node-c288() -> ()  [unwired: 2 out]
  }
  n2335 = node-c288(w3) -> ()  [unwired: 1 out]
  n2336 = call-poly <vilib>:"Close Input Device.vi"("device ID"=w21) -> ()  [unwired: 9 in, 1 out]
  n2337 = node-c288(w6) -> ()  [unwired: 1 out]
  n2338 = node-c288(w67) -> ()  [unwired: 1 out]
  n2339 = node-c288(w74) -> ()  [unwired: 1 out]
  n2340 = node-c288(w72) -> ()  [unwired: 1 out]
  n2341 = node-c288(w162) -> ()  [unwired: 1 out]
  n2342 = flat-sequence {
    tunnel: w30 -> [w9103]
    tunnel: [w9102] -> w36
    tunnel: [w9099] -> w35
    tunnel: w34 -> [_]
    tunnel: w33 -> [_]
    tunnel: w32 -> [_]
    tunnel: w31 -> [_]
    tunnel: w29 -> [w9100]
    tunnel: w36 -> [w9165]
    tunnel: w35 -> [w9164]
    frame #0 {
      w9101 = FALSE ("APD to FIFO")
      n2343 = xnode "Read/Write Control"("FPGA VI Reference In"=w9103, "error in"=w9100, "APD to FIFO"=w9101, "AI to FIFO"=w9101) -> ("FPGA VI Reference Out"=w9102:T19, "error out"=w9099:errorcluster)
    }
    frame #1 {
      n2344 = xnode "Invoke Method"("FPGA VI Reference In"=w9165, "error in"=w9164) -> ("FPGA VI Reference Out"=w9163:T19)  [unwired: 1 out]
      n2345 = xnode "Close FPGA VI Reference"("FPGA VI Reference In"=w9163) -> ()  [unwired: 1 in, 1 out]
    }
  }
